vi "UHR-Fleezers Control (host) - 10.6.vi"() -> ()   [LabVIEW 2010] (continued)
        n1249 = control-ref of="Trap Delta (MHz)"() -> (w4746:refnum<vi>)
        n1250 = Equal?(x=w4746, y=w4747) -> (x = y?=w4745:bool)
        n1251 = case shown="False" "Oscillate Set 1" {
          tunnel: w4750 -> [w4770 _]
          tunnel: [w4769 w4773] -> w4749
          tunnel: w4748 -> [w4768 w4773]
          tunnel: w4745 -> [w4753 _]
          frame False {
            n1252 = local read "BD 1 Frequency 2 (MHz)"() -> (w4757:dbl)
            n1253 = local read "BD 1 Frequency 1 (MHz)"() -> (w4755:dbl)
            n1254 = Subtract(x=w4757, y="Trap Delta (MHz)") -> (x-y=w4754:dbl)
            n1255 = Select(t=w4754, s=w4753, f=w4755) -> (s? t:f=w4752:dbl)
            n1256 = local read "Y RF Frequency Limits (MHz)"() -> (w4758:T16)
            n1257 = local read "X RF Frequency Limits (MHz)"() -> (w4759:T16)
            n1258 = local read "BD 1 Frequency 3 (MHz)"() -> (w4771:dbl)
            n1259 = local write "BD 1 Frequency 1 (MHz)"(w4752) -> ()
            n1260 = local read "BD 2 Frequency 1 (MHz)"() -> (w4762:dbl)
            n1261 = local read "BD 2 Frequency 2 (MHz)"() -> (w4761:dbl)
            n1262 = local read "BD 2 Frequency 3 (MHz)"() -> (w4772:dbl)
            n1263 = call "set RF board frequency - interlace.vi"("Board 2 Frequency Limits"=w4758, "Board 1 Frequency Limits"=w4759, "error in"=w4768, "FPGA VI Reference In"=w4770, "Board 2 Frequency 3 (MHz)"=w4772, "Board 1 Frequency 3 (MHz)"=w4771, "Board 2 Frequency 2 (MHz)"=w4761, "Board 2 Frequency 1 (MHz)"=w4762, "Board 1 Frequency 2 (MHz)"=w4757, "Board 1 Frequency 1  (MHz)"=w4752) -> ("error out"=w4769:errorcluster)  [unwired: 1 out]
            n1264 = Subtract(x=w4762, y=w4761) -> (x-y=w4766:dbl)
            n1265 = Subtract(x=w4752, y=w4757) -> (x-y=w4767:dbl)
            n1266 = Square(x=w4766) -> (x^2=w4764:dbl)
            n1267 = Square(x=w4767) -> (x^2=w4765:dbl)
            n1268 = Add(x=w4765, y=w4764) -> (x+y=w4763:dbl)
            n1269 = Square Root(x=w4763) -> (sqrt(x)=w4760:dbl)
            n1270 = local write "Trap Delta (MHz)"(w4760) -> ()
            n1271 = property on="Initial delta (MHz)" class="DigNum (strict)"("Val(Sgnl)"=w4760) -> ()  [unwired: 2 in, 2 out]
          }
          frame True {
          }
        }
      }
      event "Round T1 X": Value Change {
        n1272 = event-data() -> ()  [unwired: 7 out]
        n1273 = local read "BD 1 Frequency 1 (MHz)"() -> (w4776:dbl)
        n1274 = Round To Nearest(number=w4776) -> (nearest integer value=w4775:dbl)
        n1275 = property on="BD 1 Frequency 1 (MHz)" class="DigNum (strict)"("Val(Sgnl)"=w4775) -> ()  [unwired: 2 in, 2 out]
      }
      event "Restart RF": Value Change {
        n1276 = event-data() -> ()  [unwired: 7 out]
        n1277 = xnode "Read/Write Control"("FPGA VI Reference In"=w4814, "error in"=w4809, "FPGA Controls  RF Box"=FALSE) -> ("FPGA VI Reference Out"=w4813:T20, "error out"=w4808:errorcluster)
        n1278 = local read "Y RF Amplitude Limits (%)"() -> (w4789:T16)
        n1279 = local read "X RF Amplitude Limits (%)"() -> (w4790:T16)
        n1280 = local read "X RF Frequency Limits (MHz)"() -> (w4792:T16)
        n1281 = local read "Y RF Frequency Limits (MHz)"() -> (w4791:T16)
        n1282 = xnode "Read/Write Control"("FPGA VI Reference In"=w4813, "error in"=w4808, "Direct RF Box  Communication"=TRUE) -> ("FPGA VI Reference Out"=w4812:T20, "error out"=w4807:errorcluster)
        n1283 = local read "BD 2 Frequency 3 (MHz)"() -> (w4799:dbl)
        n1284 = local read "BD 2 Frequency 2 (MHz)"() -> (w4800:dbl)
        n1285 = local read "BD 1 Frequency 3 (MHz)"() -> (w4803:dbl)
        n1286 = local read "BD 1 Frequency 1 (MHz)"() -> (w4804:dbl)
        n1287 = local read "BD 2 Frequency 1 (MHz)"() -> (w4801:dbl)
        n1288 = local read "BD 1 Frequency 2 (MHz)"() -> (w4802:dbl)
        n1289 = call "Initialize RF boards - interlace 3.vi"("error in"=w4807, "FPGA VI Reference In"=w4812) -> ("error out"=w4806:errorcluster, "FPGA VI Reference Out"=w4811:T20)
        n1290 = local read "BD 2 Amplitude 2 (%)"() -> (w4794:dbl)
        n1291 = local read "BD 2 Amplitude 1 (%)"() -> (w4795:dbl)
        n1292 = local read "BD 2 Amplitude 3 (%)"() -> (w4793:dbl)
        n1293 = local read "BD 1 Amplitude 3 (%)"() -> (w4798:dbl)
        n1294 = local read "BD 1 Amplitude 1 (%)"() -> (w4797:dbl)
        n1295 = local read "BD 1 Amplitude 2 (%)"() -> (w4796:dbl)
        n1296 = call "set RF board frequency - interlace.vi"("Board 2 Frequency Limits"=w4791, "Board 1 Frequency Limits"=w4792, "error in"=w4806, "FPGA VI Reference In"=w4811, "Board 2 Frequency 3 (MHz)"=w4799, "Board 1 Frequency 3 (MHz)"=w4803, "Board 2 Frequency 2 (MHz)"=w4800, "Board 2 Frequency 1 (MHz)"=w4801, "Board 1 Frequency 2 (MHz)"=w4802, "Board 1 Frequency 1  (MHz)"=w4804) -> ("error out"=w4805:errorcluster, "FPGA VI Reference Out"=w4810:T20)
        n1297 = call "set RF board amplitude - interlace.vi"("Board 2 Amplitude Limits"=w4789, "Board 1 Amplitude Limits"=w4790, "error in"=w4805, "FPGA VI Reference In"=w4810, "Board 2 Amplitude 3 (%)"=w4793, "Board 1 Amplitude 3 (%)"=w4798, "Board 2 Amplitude 2 (%)"=w4794, "Board 2 Amplitude 1 (%)"=w4795, "Board 1 Amplitude 2 (%)"=w4796, "Board 1 Amplitude 1 (%)"=w4797) -> ("error out"=w4782:errorcluster, "FPGA VI Reference Out"=w4786:T20)
        n1298 = xnode "Read/Write Control"("FPGA VI Reference In"=w4786, "error in"=w4782, "Direct RF Box  Communication"=FALSE) -> ("FPGA VI Reference Out"=w4785:T20, "error out"=w4784:errorcluster)
        n1299 = flat-sequence {
          tunnel: w4784 -> [w4815]
          tunnel: [w4815] -> w4783
          frame #0 {
            n1300 = Wait (ms)(milliseconds to wait=u32 50) -> ()  [unwired: 1 out]
          }
        }
        n1301 = xnode "Read/Write Control"("FPGA VI Reference In"=w4785, "error in"=w4783, "FPGA Controls  RF Box"=TRUE) -> ("error out"=w4778:errorcluster)  [unwired: 1 out]
        n1302 = property on="Restart RF" class="Bool (strict)"(error in=w4778, "Value"=FALSE ("Restart RF")) -> (error out=w4777:errorcluster)  [unwired: 1 in, 1 out]
      }
      event "Round T2 X": Value Change {
        n1303 = event-data() -> ()  [unwired: 7 out]
        n1304 = local read "BD 1 Frequency 2 (MHz)"() -> (w4970:dbl)
        n1305 = Round To Nearest(number=w4970) -> (nearest integer value=w4969:dbl)
        n1306 = property on="BD 1 Frequency 2 (MHz)" class="DigNum (strict)"("Val(Sgnl)"=w4969) -> ()  [unwired: 2 in, 2 out]
      }
      event "Stop All": Value Change {
        n1307 = event-data() -> ()  [unwired: 7 out]
        n1308 = local read "Stop All"() -> (w4972:bool)
      }
      event "Delayed Interlace Start": Value Change {
        n1309 = event-data() -> ()  [unwired: 7 out]
        n1310 = flat-sequence {
          frame #0 {
            n1311 = Multiply(x="Delay to Interlace (s)", y=1000.0) -> (x*y=w4975:dbl)
            n1312 = Wait (ms)(milliseconds to wait=w4975) -> ()  [unwired: 1 out]
          }
          frame #1 {
            n1313 = property on="Green laser mode" class="RadioBtnsControl (strict)"("Val(Sgnl)"=enum32{"Laser ON", "Laser OFF", "Interlace"}."Interlace" ("Value (Signaling)")) -> ()  [unwired: 2 in, 2 out]
          }
        }
      }
      event "BD 1 Amplitude 1 (%)", "BD 1 Amplitude 2 (%)", "BD 1 Amplitude 3 (%)", "BD 2 Amplitude 1 (%)", "BD 2 Amplitude 2 (%)", "BD 2 Amplitude 3 (%)", "Trap 1 ON", "Trap 2 ON", "Trap 3 ON", "Feedback On/Off", "All FB On/Off": Value Change {
        w4999 = i16 1 ("f")
        n1314 = event-data() -> ()  [unwired: 7 out]
        n1315 = local write "Trap 1 (ON/OFF)"("Trap 1 ON") -> ()
        n1316 = local write "Trap 2 (ON/OFF)"("Trap 2 ON") -> ()
        n1317 = Boolean To (0,1)(Boolean="Trap 3 ON") -> (0, 1=w5000:i16)
        n1318 = Boolean To (0,1)(Boolean="Trap 1 ON") -> (0, 1=w5001:i16)
        n1319 = Boolean To (0,1)(Boolean="Trap 2 ON") -> (0, 1=w5002:i16)
        n1320 = Select(t=w5002, s="Trap ON/OFF X or Y Amp?", f=w4999) -> (s? t:f=w4997:i16)
        n1321 = Select(t=w5001, s="Trap ON/OFF X or Y Amp?", f=w4999) -> (s? t:f=w4998:i16)
        n1322 = Select(t=w5000, s="Trap ON/OFF X or Y Amp?", f=w4999) -> (s? t:f=w4996:i16)
        n1323 = Select(t=w4999, s="Trap ON/OFF X or Y Amp?", f=w5002) -> (s? t:f=w4994:i16)
        n1324 = Select(t=w4999, s="Trap ON/OFF X or Y Amp?", f=w5001) -> (s? t:f=w4995:i16)
        n1325 = Select(t=w4999, s="Trap ON/OFF X or Y Amp?", f=w5000) -> (s? t:f=w4993:i16)
        n1326 = And(x="All FB On/Off", y="Feedback On/Off") -> (x .and. y?=w4991:cluster{"Set 1":bool, "Set 2":bool})
        n1327 = local read "BD 1 Amplitude 1 (%)"() -> (w5011:dbl)
        n1328 = local read "BD 1 Amplitude 2 (%)"() -> (w5010:dbl)
        n1329 = local read "BD 1 Amplitude 3 (%)"() -> (w5009:dbl)
        n1330 = Unbundle By Name(w4991) -> ("Set 1"=w4986:bool, "Set 2"=w4983:bool)
        n1331 = local read "Y RF Amplitude Limits (%)"() -> (w4979:T16)
        n1332 = local read "X RF Amplitude Limits (%)"() -> (w4980:T16)
        n1333 = local read "BD 2 Amplitude 1 (%)"() -> (w5012:dbl)
        n1334 = local read "BD 2 Amplitude 2 (%)"() -> (w5013:dbl)
        n1335 = local read "BD 2 Amplitude 3 (%)"() -> (w5014:dbl)
        n1336 = And(x="Trap 2 ON", y=w4983) -> (x .and. y?=w4981:bool)
        n1337 = And(x="Trap 1 ON", y=w4986) -> (x .and. y?=w4984:bool)
        n1338 = Multiply(x=w4998, y=w5011) -> (x*y=w5006:dbl)
        n1339 = Multiply(x=w5010, y=w4997) -> (x*y=w5004:dbl)
        n1340 = Multiply(x=w5009, y=w4996) -> (x*y=w5005:dbl)
        n1341 = Multiply(x=w5012, y=w4995) -> (x*y=w5015:dbl)
        n1342 = Multiply(x=w5013, y=w4994) -> (x*y=w5016:dbl)
        n1343 = Multiply(x=w5014, y=w4993) -> (x*y=w5017:dbl)
        n1344 = call "set RF board amplitude - interlace.vi"("Board 2 Amplitude Limits"=w4979, "Board 1 Amplitude Limits"=w4980, "error in"=w5007, "FPGA VI Reference In"=w5008, "Board 2 Amplitude 3 (%)"=w5017, "Board 1 Amplitude 3 (%)"=w5005, "Board 2 Amplitude 2 (%)"=w5016, "Board 2 Amplitude 1 (%)"=w5015, "Board 1 Amplitude 2 (%)"=w5004, "Board 1 Amplitude 1 (%)"=w5006) -> ("error out"=w4988:errorcluster, "FPGA VI Reference Out"=w4989:T20)
        n1345 = xnode "Read/Write Control"("FPGA VI Reference In"=w4989, "error in"=w4988, "FB On/Off Set 1"=w4984, "FB On/Off Set 2"=w4981) -> ("error out"=w4987:errorcluster)  [unwired: 1 out]
      }
      event "Load parameters": Value Change {
        n1346 = event-data() -> ()  [unwired: 7 out]
        n1347 = property on="Saved AOD Raster Scan Parameter Sets" class="Arr (strict)"() -> ("Index Values"=w5087:u32[])  [unwired: 2 in, 2 out]
        n1348 = Index Array(array=w5087, index=0) -> (element=w5084:u32)
        n1349 = local write "Load parameters"(FALSE ("Load parameters")) -> ()
        n1350 = Index Array(array="Saved AOD Raster Scan Parameter Sets", index=w5084) -> (element=w5083:T48)
        n1351 = Unbundle By Name(w5083) -> ("Scan Range AOD (nm) 2"=w5082:dbl, "Step Size AOD (nm) 2"=w5081:dbl, "Scan Speed AOD (nm/s) 2"=w5080:dbl, "Number of scans (AOD) 2"=w5079:u16)
        n1352 = flat-sequence {
          tunnel: w5082 -> [w5090]
          tunnel: w5081 -> [w5089]
          tunnel: w5080 -> [w5088]
          tunnel: w5079 -> [w5091]
          frame #0 {
            n1353 = local write "Scan Speed (nm/s)"(w5088) -> ()
            n1354 = local write "Scan Range (nm)"(w5090) -> ()
            n1355 = local write "Step Size (nm)"(w5089) -> ()
          }
          frame #1 {
            n1356 = property on="Number of F/B Scans (AOD)" class="DigNum (strict)"("Val(Sgnl)"=w5091) -> ()  [unwired: 2 in, 2 out]
          }
        }
      }
      event "Trap 1 (ON/OFF)", "Trap 2 (ON/OFF)": Value Change {
        n1357 = event-data() -> ()  [unwired: 7 out]
        n1358 = property on="Trap 2 ON" class="Bool (strict)"("Val(Sgnl)"="Trap 2 (ON/OFF)") -> ()  [unwired: 2 in, 2 out]
        n1359 = property on="Trap 1 ON" class="Bool (strict)"("Val(Sgnl)"="Trap 1 (ON/OFF)") -> ()  [unwired: 2 in, 2 out]
      }
      event "DIO count 1 (ticks)", "DIO count 2 (ticks)", "DIO count 3 (ticks)", "Interlace", "Number Interlace Sets", "Not-Interlacing Set": Value Change {
        n1360 = event-data() -> ()  [unwired: 7 out]
        n1361 = local read "DIO count 3 (ticks)"() -> (w5104:u32)
        n1362 = local read "DIO count 1 (ticks)"() -> (w5106:u32)
        n1363 = local read "DIO count 2 (ticks)"() -> (w5105:u32)
        n1364 = To Unsigned Byte Integer(number="Not-Interlacing Set") -> (unsigned 8bit integer=w5095:u8)
        n1365 = Add(x=w5095, y=u8 1) -> (x+y=w5099:u8)
        n1366 = xnode "Read/Write Control"("FPGA VI Reference In"=w5110, "error in"=w5108, "DIO count 1 (ticks)"=w5106, "DIO count 2 (ticks)"=w5105, "DIO count 3 (ticks)"=w5104, "Interlace ON/OFF"="Interlace", "Number Interlace Cycles"="Number Interlace Sets", "Interlace Off Parameters"=w5099) -> ("error out"=w5109:errorcluster)  [unwired: 1 out]
        n1367 = Build Array(w5106, w5105, w5104) -> (w5097:u32[])
        n1368 = Split 1D Array(array=w5097, index="Number Interlace Sets") -> (first subarray=w5107:u32[])  [unwired: 1 out]
        n1369 = Index Array(array=w5097, index=w5095) -> (element=w5096:u32)
        n1370 = Add Array Elements(numeric array=w5107) -> (sum=w5101:u32)
        n1371 = Select(t=w5101, s="Interlace", f=w5096) -> (s? t:f=→"Total Counts (ticks)":u32)
      }
      event "Reset Feedback": Value Change {
        n1372 = event-data() -> ()  [unwired: 7 out]
        n1373 = Unbundle By Name("Reset Feedback") -> ("Set 1"=w5252:bool, "Set 2"=w5251:bool)
        n1374 = xnode "Read/Write Control"("FPGA VI Reference In"=w5254, "error in"=w5249, "FB Reset Set 1"=w5252, "FB Reset Set 2"=w5251) -> ("error out"=w5250:errorcluster)  [unwired: 1 out]
      }
      event "PID Gains": Value Change {
        n1375 = event-data() -> ()  [unwired: 7 out]
        n1376 = Unbundle By Name("PID Gains") -> ("Set 1"=w5317:T14, "Set 2"=w5316:T14)
        n1377 = xnode "Read/Write Control"("FPGA VI Reference In"=w5318, "error in"=w5314, "FB Gains Set 1"=w5317, "FB Gains Set 2"=w5316) -> ("error out"=w5315:errorcluster)  [unwired: 1 out]
      }
      event "AI2 to Setpoint", "Trap Intensity\nSetpoints (V)": Value Change {
        n1378 = event-data() -> ()  [unwired: 7 out]
        n1379 = xnode "Read/Write Control"("FPGA VI Reference In"=w5393, "error in"=w5389) -> ("FPGA VI Reference Out"=w5392:T20, "error out"=w5391:errorcluster, "AI2 Y Sum Set 1"=w5400:i16, "AI2 Y Sum Set 2"=w5399:i16)
        n1380 = Cluster To Array(cluster="AI2 to Setpoint") -> (array=w5403:bool[])
        n1381 = local read "AI2 (V)"() -> (w5401:cluster{"Set 1":dbl, "Set 2":dbl})
        n1382 = Or Array Elements(Boolean array=w5403) -> (logical OR=w5404:bool)
        n1383 = Bundle By Name(cluster=w5401, "Set 1"=w5400, "Set 2"=w5399) -> (w5398:cluster{"Set 1":dbl, "Set 2":dbl})
        n1384 = Divide(x=w5398, y=3276.7) -> (x/y=w5397:cluster{"Set 1":dbl, "Set 2":dbl})
        "AI2 (V)" <- w5397
        n1385 = case shown="True" w5404 {
          tunnel: [w5468 w5485] -> w5396
          tunnel: "AI2 to Setpoint" -> [_ w5481]
          tunnel: "Trap Intensity\nSetpoints (V)" -> [w5469 w5484]
          tunnel: w5397 -> [_ w5478]
          frame False {
            n1386 = Multiply(x=3276.7, y=w5469) -> (x*y=w5470:cluster{"Set 1":dbl, "Set 2":dbl})
            n1387 = To Word Integer(number=w5470) -> (16bit integer=w5468:cluster{"Set 1":i16, "Set 2":i16})
          }
          frame True {
            n1388 = Unbundle By Name(w5478) -> ("Set 1"=w5477:dbl, "Set 2"=w5476:dbl)
            n1389 = Unbundle By Name(w5484) -> ("Set 1"=w5483:dbl, "Set 2"=w5482:dbl)
            n1390 = Unbundle By Name(w5481) -> ("Set 1"=w5480:bool, "Set 2"=w5479:bool)
            n1391 = Select(t=w5477, s=w5480, f=w5483) -> (s? t:f=w5475:dbl)
            n1392 = Select(t=w5476, s=w5479, f=w5482) -> (s? t:f=w5474:dbl)
            n1393 = Bundle By Name(cluster=w5484, "Set 1"=w5475, "Set 2"=w5474) -> (w5472:cluster{"Set 1":dbl, "Set 2":dbl})
            n1394 = local write "Trap Intensity\nSetpoints (V)"(w5472) -> ()
            n1395 = Multiply(x=3276.7, y=w5472) -> (x*y=w5473:cluster{"Set 1":dbl, "Set 2":dbl})
            n1396 = To Word Integer(number=w5473) -> (16bit integer=w5485:cluster{"Set 1":i16, "Set 2":i16})
          }
        }
        n1397 = Unbundle By Name(w5396) -> ("Set 1"=w5395:i16, "Set 2"=w5394:i16)
        n1398 = xnode "Read/Write Control"("FPGA VI Reference In"=w5392, "error in"=w5391, "FB Setpoint Set 1"=w5395, "FB Setpoint Set 2"=w5394) -> ("error out"=w5390:errorcluster)  [unwired: 1 out]
      }
      event "Invert GI": Value Change {
        n1399 = event-data() -> ()  [unwired: 7 out]
        n1400 = xnode "Read/Write Control"("FPGA VI Reference In"=w5547, "error in"=w5545, "Invert GI"="Invert GI", "Invert GI 2"="Invert GI") -> ("error out"=w5546:errorcluster)  [unwired: 1 out]
      }
      event "Green FB Setpoint (mV)", "Green FB Gains", "Green FB On/Off", "Current When FB OFF (%)", "Green int current ON count adj": Value Change {
        n1401 = event-data() -> ()  [unwired: 7 out]
        n1402 = local read "Green FB Setpoint (mV)"() -> (w5613:dbl)
        n1403 = local read "Current When FB OFF (%)"() -> (w5616:dbl)
        n1404 = Multiply(x=w5613, y=3.2767) -> (x*y=w5612:dbl)
        n1405 = Multiply(x=w5616, y=655.35) -> (x*y=w5617:dbl)
        n1406 = To Unsigned Word Integer(number=w5617) -> (unsigned 16bit integer=w5615:u16)
        n1407 = local read "Green int current ON count adj"() -> (w5620:u32)
        n1408 = local read "Green FB Gains"() -> (w5619:T14)
        n1409 = local read "Green Laser ON/Interlacing"() -> (w5610:bool)
        n1410 = local read "Green laser mode"() -> (w5609:enum32{"Laser ON", "Laser OFF", "Interlace"})
        n1411 = local read "Green FB On/Off"() -> (w5621:bool)
        n1412 = Equal?(x=w5609, y=enum32{"Laser ON", "Laser OFF", "Interlace"}."Interlace") -> (x = y?=w5607:bool)
        n1413 = Compound Arithmetic op=AND(w5607, w5621, w5610) -> (w5611:bool)
        n1414 = xnode "Read/Write Control"("FPGA VI Reference In"=w5624, "error in"=w5623, "Green FB Setpoint"=w5612, "Green FB On/Off"=w5611, "Current Out"=w5615, "Green int current ON count adj"=w5620, "Green FB Gains"=w5619) -> ("error out"=w5622:errorcluster)  [unwired: 1 out]
      }
      event "Green laser mode", "Green Laser ON/Interlacing": Value Change {
        n1415 = event-data() -> ()  [unwired: 7 out]
        n1416 = case shown="True" "Green Laser ON/Interlacing" {
          tunnel: "Green laser mode" -> [_ w5762]
          tunnel: [enum32{"Laser ON", "Laser OFF", "Interlace"}."Laser OFF" ("Green laser mode") w5762] -> w5750
          tunnel: [FALSE w5758] -> w5749
          frame False {
          }
          frame True {
            n1417 = local read "Green FB On/Off"() -> (w5759:bool)
            n1418 = Equal?(x=w5762, y=enum32{"Laser ON", "Laser OFF", "Interlace"}."Interlace") -> (x = y?=w5760:bool)
            n1419 = And(x=w5760, y=w5759) -> (x .and. y?=w5758:bool)
          }
        }
        n1420 = xnode "Read/Write Control"("FPGA VI Reference In"=w5755, "error in"=w5753, "Operating Mode"=w5750, "Operating Mode 2"=w5750, "Green FB On/Off"=w5749) -> ("error out"=w5754:errorcluster)  [unwired: 1 out]
      }
      event "Use mouse to move stage\n(press mouse wheel to quit)": Value Change {
        n1421 = event-data() -> ()  [unwired: 7 out]
      }
      event "- phase (APD 1 Gate)", "+ phase (APD 1 Gate)": Value Change {
        n1422 = event-data() -> ()  [unwired: 7 out]
        n1423 = local read "Phase Adj. (APD 1 Gate)"() -> (w5841:i16)
        n1424 = Negate(x=w5841) -> (-x=w5849:i16)
        n1425 = Select(t=w5849, s="- phase (APD 1 Gate)", f=w5841) -> (s? t:f=w5848:i16)
        n1426 = Or(x="- phase (APD 1 Gate)", y="+ phase (APD 1 Gate)") -> (x .or. y?=w5844:bool)
        n1427 = xnode "Read/Write Control"("FPGA VI Reference In"=w5851, "error in"=w5850, "Phase count adjustment (APD 1 Gate)"=w5848) -> ("FPGA VI Reference Out"=w5846:T20, "error out"=w5847:errorcluster)
        n1428 = xnode "Read/Write Control"("FPGA VI Reference In"=w5846, "error in"=w5847, "+ phase (APD 1 Gate)"=w5844) -> ("error out"=w5845:errorcluster)  [unwired: 1 out]
      }
      event "+ phase (APD 2 Gate)", "- phase (APD 2 Gate)": Value Change {
        n1429 = event-data() -> ()  [unwired: 7 out]
        n1430 = local read "Phase Adj. (APD 2 Gate)"() -> (w5927:i16)
        n1431 = Negate(x=w5927) -> (-x=w5935:i16)
        n1432 = Select(t=w5935, s="- phase (APD 2 Gate)", f=w5927) -> (s? t:f=w5934:i16)
        n1433 = Or(x="- phase (APD 2 Gate)", y="+ phase (APD 2 Gate)") -> (x .or. y?=w5930:bool)
        n1434 = xnode "Read/Write Control"("FPGA VI Reference In"=w5937, "error in"=w5936, "Phase count adjustment (APD 2 Gate)"=w5934) -> ("FPGA VI Reference Out"=w5932:T20, "error out"=w5933:errorcluster)
        n1435 = xnode "Read/Write Control"("FPGA VI Reference In"=w5932, "error in"=w5933, "+ phase (APD 2 Gate)"=w5930) -> ("error out"=w5931:errorcluster)  [unwired: 1 out]
      }
      event "Phase Adj. (APD Acq)", "+ phase (APD Acq)", "- phase (APD Acq)": Value Change {
        n1436 = event-data() -> ()  [unwired: 7 out]
        n1437 = local read "Phase Adj. (APD Acq)"() -> (w6015:i16)
        n1438 = Negate(x=w6015) -> (-x=w6021:i16)
        n1439 = Select(t=w6021, s="+ phase (APD Acq)", f=w6015) -> (s? t:f=w6020:i16)
        n1440 = Or(x="+ phase (APD Acq)", y="- phase (APD Acq)") -> (x .or. y?=w6016:bool)
        n1441 = xnode "Read/Write Control"("FPGA VI Reference In"=w6023, "error in"=w6022, "Phase Count Adjustment (APD Acq)"=w6020) -> ("FPGA VI Reference Out"=w6018:T20, "error out"=w6019:errorcluster)
        n1442 = xnode "Read/Write Control"("FPGA VI Reference In"=w6018, "error in"=w6019, "+ phase (APD Acq)"=w6016) -> ("error out"=w6017:errorcluster)  [unwired: 1 out]
      }
      event "Phase adj. (GI)", "+ phase (GI)", "- phase (GI)": Value Change {
        n1443 = event-data() -> ()  [unwired: 7 out]
        n1444 = Negate(x="Phase adj. (GI)") -> (-x=w6107:i16)
        n1445 = Select(t=w6107, s="+ phase (GI)", f="Phase adj. (GI)") -> (s? t:f=w6106:i16)
        n1446 = Or(x="+ phase (GI)", y="- phase (GI)") -> (x .or. y?=w6102:bool)
        n1447 = xnode "Read/Write Control"("FPGA VI Reference In"=w6109, "error in"=w6108, "Phase count adjustment (GI)"=w6106) -> ("FPGA VI Reference Out"=w6104:T20, "error out"=w6105:errorcluster)
        n1448 = xnode "Read/Write Control"("FPGA VI Reference In"=w6104, "error in"=w6105, "+ phase (GI)"=w6102) -> ("error out"=w6103:errorcluster)  [unwired: 1 out]
      }
      event "Phase adj. (GI) 2", "+ phase (GI) 2", "- phase (GI) 2": Value Change {
        n1449 = event-data() -> ()  [unwired: 7 out]
        n1450 = Negate(x="Phase adj. (GI) 2") -> (-x=w6193:i16)
        n1451 = Select(t=w6193, s="+ phase (GI) 2", f="Phase adj. (GI) 2") -> (s? t:f=w6192:i16)
        n1452 = Or(x="+ phase (GI) 2", y="- phase (GI) 2") -> (x .or. y?=w6188:bool)
        n1453 = xnode "Read/Write Control"("FPGA VI Reference In"=w6195, "error in"=w6194, "Phase count adjustment (GI) 2"=w6192) -> ("FPGA VI Reference Out"=w6190:T20, "error out"=w6191:errorcluster)
        n1454 = xnode "Read/Write Control"("FPGA VI Reference In"=w6190, "error in"=w6191, "+ phase (GI) 2"=w6188) -> ("error out"=w6189:errorcluster)  [unwired: 1 out]
      }
      event "Phase adj. (Green FB)", "- phase (Green FB)", "+ phase (Green FB)": Value Change {
        n1455 = event-data() -> ()  [unwired: 7 out]
        n1456 = Negate(x="Phase adj. (Green FB)") -> (-x=w6279:i16)
        n1457 = Select(t=w6279, s="+ phase (Green FB)", f="Phase adj. (Green FB)") -> (s? t:f=w6278:i16)
        n1458 = Or(x="+ phase (Green FB)", y="- phase (Green FB)") -> (x .or. y?=w6274:bool)
        n1459 = xnode "Read/Write Control"("FPGA VI Reference In"=w6281, "error in"=w6280, "Phase count adjustment (Green FB)"=w6278) -> ("FPGA VI Reference Out"=w6276:T20, "error out"=w6277:errorcluster)
        n1460 = xnode "Read/Write Control"("FPGA VI Reference In"=w6276, "error in"=w6277, "+ phase (Green FB)"=w6274) -> ("error out"=w6275:errorcluster)  [unwired: 1 out]
      }
      event "Invert APD Gate", "APD Gate ON Count", "APD Gate OFF Count", "APD Gate", "APD Integration Time (s)", "APD 1 AO Mult.", "APD 2 AO Mult.": Value Change {
        n1461 = event-data() -> ()  [unwired: 7 out]
        n1462 = local read "APD Integration Time (s)"() -> (w6357:dbl)
        n1463 = local read "APD Gate ON Count"() -> (w6370:u32)
        n1464 = local read "APD Gate OFF Count"() -> (w6369:u32)
        n1465 = local read "Invert APD Gate"() -> (w6371:bool)
        n1466 = local read "APD Gate"() -> (w6368:enum32{"ON", "OFF", "Interlace"})
        n1467 = Multiply(x=w6357, y=40000000.0) -> (x*y=w6366:dbl)
        n1468 = Reciprocal(x=w6357) -> (1/x=→"APD Acq Rate (Hz)":dbl)
        n1469 = To Unsigned Long Integer(number=w6366) -> (unsigned 32bit integer=w6365:u32)
        n1470 = local read "DMA Update Period (s)"() -> (w6358:dbl)
        n1471 = Divide(x=w6358, y=w6357) -> (x/y=w6361:dbl)
        n1472 = local read "APD 1 AO Mult."() -> (w6363:i16)
        n1473 = local read "APD 2 AO Mult."() -> (w6362:i16)
        n1474 = Multiply(x=2.0, y=w6361) -> (x*y=w6360:dbl)
        n1475 = local write "APD Samples/FIFO Acq."(w6361) -> ()
        n1476 = local write "APD Elements/DMA read"(w6360) -> ()
        n1477 = xnode "Read/Write Control"("FPGA VI Reference In"=w6374, "error in"=w6373, "Invert APD Gate"=w6371, "APD Gate ON Count"=w6370, "APD Gate OFF Count"=w6369, "APD Acq Rate Count"=w6365, "APD Gate Operating Mode"=w6368, "APD 1 AO scale factor"=w6363, "APD 2 AO scale factor"=w6362) -> ("error out"=w6372:errorcluster)  [unwired: 1 out]
      }
      event "GI Frequency, ON count", "Green FB Count", "GI Frequency, OFF count": Value Change {
        n1478 = event-data() -> ()  [unwired: 7 out]
        n1479 = xnode "Read/Write Control"("FPGA VI Reference In"=w6538, "error in"=w6536, "Green interlace ON count"="GI Frequency, ON count", "Green interlace OFF count"="GI Frequency, OFF count", "Green interlace ON count 2"="GI Frequency, ON count", "Green interlace OFF count 2"="GI Frequency, OFF count", "Green FB Count"="Green FB Count") -> ("error out"=w6537:errorcluster)  [unwired: 1 out]
      }
      event "Number of F/B Scans (AOD)", "Scan Speed (nm/s)", "Scan BD", "Initial delta (MHz)", "Step Size (nm)", "Scan Range (nm)": Value Change {
        n1480 = event-data() -> ()  [unwired: 7 out]
        n1481 = local read "BD 1 Frequency 1 (MHz)"() -> (w6701:dbl)
        n1482 = local read "AOM X Cal (nm/MHz)"() -> (w6693:dbl)
        n1483 = local read "X RF Frequency Limits (MHz)"() -> (w6705:T16)
        n1484 = local read "Y RF Frequency Limits (MHz)"() -> (w6702:T16)
        n1485 = local read "BD 2 Frequency 1 (MHz)"() -> (w6707:dbl)
        n1486 = Negate(x="Scan Range (nm)") -> (-x=w6671:dbl)
        n1487 = Divide(x=w6671, y=w6693) -> (x/y=w6675:dbl)
        n1488 = Select(t=w6705, s="Scan BD", f=w6702) -> (s? t:f=w6704:T16)
        n1489 = Select(t=w6701, s="Scan BD", f=w6707) -> (s? t:f=w6706:dbl)
        n1490 = Unbundle By Name(w6704) -> ("Maximum"=w6713:dbl, "Minimum"=w6712:dbl)
        n1491 = Add(x=w6675, y=w6706) -> (x+y=w6710:dbl)
        n1492 = Divide(x=w6671, y="Step Size (nm)") -> (x/y=w6690:dbl)
        n1493 = Divide(x="Step Size (nm)", y=w6693) -> (x/y=w6699:dbl)
        n1494 = Absolute Value(x=w6690) -> (abs(x)=w6674:dbl)
        n1495 = Sign(1:w6671) -> (0:w6672:dbl)
        n1496 = In Range and Coerce(upper limit=w6713, x=w6710, lower limit=w6712) -> (coerced(x)=w6709:dbl, In Range?=w6711:bool)
        n1497 = To Unsigned Quad Integer(1:w6674) -> (0:w6689:u64)
        "Scan steps (AOD)" <- w6689
        n1498 = call "IR AOM freq to word.vi"("Frequency In (MHz)"=w6699) -> ("Frequency Word Out (double)"=w6696:dbl)
        n1499 = Multiply(x=w6672, y=w6696) -> (x*y=w6673:dbl)
        n1500 = Subtract(x=w6710, y=w6709) -> (x-y=w6708:dbl)
        n1501 = To Quad Integer(1:w6673) -> (0:w6695:i64)
        "Incr. int (AOD)" <- w6695
        n1502 = Subtract(x=w6675, y=w6708) -> (x-y=w6694:dbl)
        "Scan Range (MHz)" <- w6694
        n1503 = Select(t=w6675, s=w6711, f=w6694) -> (s? t:f=w6714:dbl)
        n1504 = Multiply(x=w6694, y=w6693) -> (x*y=w6692:dbl)
        n1505 = Decrement(x=w6689) -> (x-1=w6741:u64)
        n1506 = Negate(x=w6692) -> (-x=w6688:dbl)
        n1507 = local write "Scan Range (nm)"(w6688) -> ()
        n1508 = Divide(x=w6714, y=w6741) -> (x/y=w6698:dbl)
        "Scan Increment (MHz)" <- w6698
        n1509 = call "IR AOM freq to word.vi"("Frequency In (MHz)"=w6698) -> ("Frequency Word Out (double)"=w6697:dbl)
        n1510 = Divide(x="Step Size (nm)", y="Scan Speed (nm/s)") -> (x/y=w6685:dbl)
        n1511 = To Quad Integer(1:w6697) -> ()  [unwired: 1 out]
        n1512 = local read "Number Interlace Sets"() -> (w6669:u8)
        n1513 = local read "AI Count (ticks)"() -> (w6670:u32)
        n1514 = local read "Total Counts (ticks)"() -> (w6668:u32)
        n1515 = local read "# Samples/trap"() -> (w6700:u32)
        n1516 = Multiply(x=w6670, y=w6669) -> (x*y=w6667:u32)
        n1517 = Divide(x=w6668, y=w6667) -> (x/y=w6666:dbl)
        n1518 = local read "AOM X Cal (nm/MHz)"() -> (w6656:dbl)
        n1519 = Select(t=w6701, s="Scan BD", f=w6707) -> (s? t:f=w6738:dbl)
        "Initial freq. (MHz)" <- w6738
        n1520 = Add(x=w6714, y=w6738) -> (x+y=→"Final freq. (MHz)":dbl)
        n1521 = Divide(x=w6668, y=40000000.0) -> (x/y=w6684:dbl)
        n1522 = Divide(x=w6685, y=w6684) -> (x/y=w6683:dbl)
        n1523 = To Unsigned Quad Integer(1:w6683) -> (0:w6658:u64)
        n1524 = Quotient & Remainder(x=w6658, y=u64 2) -> (x-y*floor(x/y)=w6662:u64)  [unwired: 1 out]
        n1525 = Equal?(x=w6662, y=u64 0) -> (x = y?=w6660:bool)
        n1526 = Decrement(x=w6658) -> (x-1=w6659:u64)
        n1527 = Select(t=w6658, s=w6660, f=w6659) -> (s? t:f=w6657:u64)
        "Cycles/step (AOD)" <- w6657
        n1528 = xnode "Read/Write Control"("FPGA VI Reference In"=w6749, "error in"=w6748, "Scan steps"=w6689, "Number of scans"="Number of F/B Scans (AOD)", "Cycles per step"=w6657, "Scan freq.  increment"=w6695, "Scan BD"="Scan BD") -> ("error out"=w6747:errorcluster)  [unwired: 1 out]
        n1529 = Multiply(x=w6689, y=w6657) -> (x*y=w6742:u64)
        n1530 = Multiply(x=w6742, y=u64 2) -> (x*y=w6665:u64)
        n1531 = Multiply(x=w6666, y=w6665) -> (x*y=w6664:dbl)
        "Data points/scan (f/b)" <- w6664
        n1532 = Multiply(x=w6664, y="Number of F/B Scans (AOD)") -> (x*y=w6745:dbl)
        "Data points/scans" <- w6745
        n1533 = Divide(x=w6745, y=w6700) -> (x/y=→"N sets should be saved":dbl)
        n1534 = Multiply(x=w6742, y=w6684) -> (x*y=w6682:dbl)
        "Time/Scan (s) (AOD)" <- w6682
        n1535 = Select(t=w6714, s="Scan BD", f=0.0) -> (s? t:f=w6739:dbl)
        n1536 = Select(t=0.0, s="Scan BD", f=w6714) -> (s? t:f=w6735:dbl)
        n1537 = local read "BD 2 Frequency 2 (MHz)"() -> (w6731:dbl)
        n1538 = local read "BD 1 Frequency 2 (MHz)"() -> (w6734:dbl)
        n1539 = Add(x=w6735, y=w6707) -> (x+y=w6732:dbl)
        n1540 = Add(x=w6701, y=w6739) -> (x+y=w6733:dbl)
        n1541 = Multiply(x=w6682, y=2.0) -> (x*y=w6681:dbl)
        n1542 = Multiply(x=w6681, y="Number of F/B Scans (AOD)") -> (x*y=w6678:dbl)
        n1543 = Divide(x=w6678, y=60.0) -> (x/y=→"Time to Finish All (min)":dbl)
        n1544 = Add(x="Trap 2 Bead Size (nm)", y="Trap 1 Bead Size (nm)") -> (x+y=w6721:dbl)
        n1545 = Divide(x=w6721, y=2.0) -> (x/y=w6716:dbl)
        n1546 = local read "Initial delta (MHz)"() -> (w6718:dbl)
        n1547 = Subtract(x=w6732, y=w6731) -> (x-y=w6729:dbl)
        n1548 = Subtract(x=w6733, y=w6734) -> (x-y=w6730:dbl)
        n1549 = Square(x=w6729) -> (x^2=w6728:dbl)
        n1550 = Square(x=w6730) -> (x^2=w6727:dbl)
        n1551 = Add(x=w6727, y=w6728) -> (x+y=w6726:dbl)
        n1552 = Square Root(x=w6726) -> (sqrt(x)=w6725:dbl)
        "Final delta (MHz)" <- w6725
        n1553 = Multiply(x=w6656, y=w6725) -> (x*y=w6724:dbl)
        n1554 = Multiply(x=w6718, y=w6656) -> (x*y=w6717:dbl)
        n1555 = Subtract(x=w6717, y=w6716) -> (x-y=→"Initial sep (nm)":dbl)
        n1556 = Subtract(x=w6724, y=w6716) -> (x-y=→"Final sep (nm)":dbl)
      }
      event "Freq or Amp switch first", "Swap F1 and F2", "Freq switch delay", "Amp switch delay": Value Change {
        n1557 = event-data() -> ()  [unwired: 7 out]
        n1558 = local read "Freq or Amp switch first"() -> (w6886:bool)
        n1559 = local read "Amp switch delay"() -> (w6887:u16)
        n1560 = local read "Freq switch delay"() -> (w6889:u16)
        n1561 = local read "Swap F1 and F2"() -> (w6888:bool)
        n1562 = xnode "Read/Write Control"("FPGA VI Reference In"=w6892, "error in"=w6891, "Freq switch delay"=w6889, "Swap F1 and F2"=w6888, "Amp switch delay"=w6887, "Freq or Amp switch first"=w6886) -> ("error out"=w6890:errorcluster)  [unwired: 1 out]
      }
      event "Scan steps (MCL)", "Number of scans (MCL)", "Scan Range (V)\n(of steps)", "2D or 1D Scan", "N APD Samp/step", "Fast Scan Dir", "Continuous MCL Scanning", "Scan lines (y)": Value Change {
        w6993 = 32767.0 ("y")
        n1563 = event-data() -> ()  [unwired: 7 out]
        n1564 = Select(t="Scan lines (y)", s="2D or 1D Scan", f="Number of scans (MCL)") -> (s? t:f=w6998:u64)
        n1565 = Decrement(x="Scan steps (MCL)") -> (x-1=w7014:u64)
        n1566 = Divide(x="Scan Range (V)\n(of steps)", y=w7014) -> (x/y=w7013:dbl)
        "Desired Scan Incr (V)" <- w7013
        n1567 = local read "APD Integration Time (s)"() -> (w7006:dbl)
        n1568 = Multiply(x=w7013, y=w6993) -> (x*y=w7022:dbl)
        n1569 = Divide(x=w7022, y=10.0) -> (x/y=w7012:dbl)
        "Desired incr (int)" <- w7012
        n1570 = local read "Update Count (MCL)"() -> (w7018:u32)
        n1571 = Round Toward -Infinity(1:w7012) -> (0:w7021:dbl)
        n1572 = To Word Integer(number=w7021) -> (16bit integer=w6996:i16)
        "Actual Incr. int (MCL)" <- w6996
        n1573 = Multiply(x=w7006, y=40000000.0) -> (x*y=w7019:dbl)
        n1574 = Divide(x=w7019, y=w7018) -> (x/y=w7017:dbl)
        n1575 = Multiply(x=i16 10, y=w6996) -> (x*y=w6994:i16)
        n1576 = Multiply(x="N APD Samp/step", y=w7017) -> (x*y=w7016:dbl)
        "Cycles/step (MCL)" <- w7016
        n1577 = Divide(x=w6994, y=w6993) -> (x/y=→"Actual MCL Inc (V)":dbl)
        n1578 = Multiply(x="N APD Samp/step", y="Scan steps (MCL)") -> (x*y=w7008:dbl)
        n1579 = local read "APD Samples/FIFO Acq."() -> (w7005:dbl)
        n1580 = Multiply(x=w7008, y=u64 2) -> (x*y=w7007:dbl)
        "Data points/scan (f+b)" <- w7007
        n1581 = Multiply(x=w7007, y=w6998) -> (x*y=w7025:dbl)
        "Data points/scans (MCL)" <- w7025
        n1582 = Multiply(x=w7006, y=w7007) -> (x*y=w6999:dbl)
        "Time/f+b scan (s) (MCL)" <- w6999
        n1583 = Divide(x=w7025, y=w7005) -> (x/y=→"N sets should be saved (MCL)":dbl)
        n1584 = Multiply(x=w6999, y=w6998) -> (x*y=→"Total Time (s)":dbl)
        n1585 = Not(x="Fast Scan Dir") -> (.not. x?=w7003:bool)
        n1586 = xnode "Read/Write Control"("FPGA VI Reference In"=w7029, "error in"=w7028, "Scan steps (MCL)"="Scan steps (MCL)", "Number of scans (MCL)"=w6998, "Cycles per step (MCL)"=w7016, "Scan freq.  increment (MCL)"=w6996, "1D or 2D Scan?"="2D or 1D Scan", "MCL Scan Axis"=w7003, "Cont. Scan (MCL)"="Continuous MCL Scanning") -> ("error out"=w7027:errorcluster)  [unwired: 1 out]
      }
      event Key Down {
        n1587 = event-data() -> ("VKey"=w7203:T49)  [unwired: 10 out]
        n1588 = local read "z nudge increment (um)"() -> (w7202:dbl)
        n1589 = case shown="\"F5\"" w7203 {
          tunnel: "lateral step size (mm)" -> [w7206 w7211 w7216 w7224 _ _ _ _ _ _ _ _ _ _ _ _ _ _ _ _ _ _ _ _ _ _ _ _ _ _ _ _ _ _ _ _ _ _ _ _ _ _ _ _ _ _ _ _ _ _ _ _ _ _ _ _]
          tunnel: w7202 -> [_ _ _ _ w7227 w7234 _ _ _ _ _ _ _ _ _ _ _ _ _ _ _ _ _ _ _ _ _ _ _ _ _ _ _ _ _ _ _ _ _ _ _ _ _ _ _ _ _ _ _ _ _ _ _ _ _ _]
          frame "Up" {
            w7208 = 0.0 ("element")
            n1590 = Negate(x=w7206) -> (-x=w7205:dbl)
            n1591 = Build Array(w7208, w7205, w7208) -> (w7207:dbl[])
            n1592 = call "CONEX_FUNCTIONAL_GLOBAL.vi"("Axis"=enum16{"X", "Y", "Z", "XY", "XZ", "YZ", "XYZ"}."Y", "Position"=w7207, "Command"=T23."REL MOVE") -> ()  [unwired: 6 in, 3 out]
          }
          frame "Down" {
            w7213 = 0.0 ("element")
            n1593 = Build Array(w7213, w7211, w7213) -> (w7212:dbl[])
            n1594 = call "CONEX_FUNCTIONAL_GLOBAL.vi"("Axis"=enum16{"X", "Y", "Z", "XY", "XZ", "YZ", "XYZ"}."Y", "Position"=w7212, "Command"=T23."REL MOVE") -> ()  [unwired: 6 in, 3 out]
          }
          frame "Left" {
            w7217 = 0.0 ("element")
            n1595 = Build Array(w7216, w7217, w7217) -> (w7218:dbl[])
            n1596 = call "CONEX_FUNCTIONAL_GLOBAL.vi"("Axis"=enum16{"X", "Y", "Z", "XY", "XZ", "YZ", "XYZ"}."X", "Position"=w7218, "Command"=T23."REL MOVE") -> ()  [unwired: 6 in, 3 out]
          }
          frame "Right" {
            w7222 = 0.0 ("element")
            n1597 = Negate(x=w7224) -> (-x=w7223:dbl)
            n1598 = Build Array(w7223, w7222, w7222) -> (w7221:dbl[])
            n1599 = call "CONEX_FUNCTIONAL_GLOBAL.vi"("Axis"=enum16{"X", "Y", "Z", "XY", "XZ", "YZ", "XYZ"}."X", "Position"=w7221, "Command"=T23."REL MOVE") -> ()  [unwired: 6 in, 3 out]
          }
          frame "PageUp" {
            w7231 = 0.0 ("element")
            n1600 = Divide(x=w7227, y=1000.0) -> (x/y=w7229:dbl)
            n1601 = Build Array(w7231, w7231, w7229) -> (w7230:dbl[])
            n1602 = call "CONEX_FUNCTIONAL_GLOBAL.vi"("Axis"=enum16{"X", "Y", "Z", "XY", "XZ", "YZ", "XYZ"}."Z", "Position"=w7230, "Command"=T23."REL MOVE") -> ()  [unwired: 6 in, 3 out]
          }
          frame "PageDown" {
            w7238 = 0.0 ("element")
            n1603 = Divide(x=w7234, y=-1000.0) -> (x/y=w7236:dbl)
            n1604 = Build Array(w7238, w7238, w7236) -> (w7237:dbl[])
            n1605 = call "CONEX_FUNCTIONAL_GLOBAL.vi"("Axis"=enum16{"X", "Y", "Z", "XY", "XZ", "YZ", "XYZ"}."Z", "Position"=w7237, "Command"=T23."REL MOVE") -> ()  [unwired: 6 in, 3 out]
          }
          frame Default {
          }
          frame "Insert" {
          }
          frame "Delete" {
          }
          frame "Home" {
          }
          frame "End" {
          }
          frame "Escape" {
          }
          frame "Help" {
          }
          frame "Pause" {
          }
          frame "ScrollLock" {
          }
          frame "F1" {
          }
          frame "F2" {
          }
          frame "F3" {
          }
          frame "F4" {
          }
          frame "F5" {
            n1606 = local read "Inject Top"() -> (w7242:bool)
            n1607 = Not(x=w7242) -> (.not. x?=w7241:bool)
            n1608 = property on="Inject Top" class="Bool (strict)"("Val(Sgnl)"=w7241) -> ()  [unwired: 2 in, 2 out]
          }
          frame "F6" {
          }
          frame "F7" {
          }
          frame "F8" {
          }
          frame "F9" {
            n1609 = local read "Trap 1 (ON/OFF)"() -> (w7244:bool)
            n1610 = Not(x=w7244) -> (.not. x?=w7243:bool)
            n1611 = property on="Trap 1 (ON/OFF)" class="Bool (strict)"("Val(Sgnl)"=w7243) -> ()  [unwired: 2 in, 2 out]
          }
          frame "F10" {
            n1612 = local read "Trap 2 (ON/OFF)"() -> (w7246:bool)
            n1613 = Not(x=w7246) -> (.not. x?=w7245:bool)
            n1614 = property on="Trap 2 (ON/OFF)" class="Bool (strict)"("Val(Sgnl)"=w7245) -> ()  [unwired: 2 in, 2 out]
          }
          frame "F11" {
            n1615 = local read "Sample Channel Flow"() -> (w7248:bool)
            n1616 = Not(x=w7248) -> (.not. x?=w7247:bool)
            n1617 = case shown="True" w7247 {
              frame False {
              }
              frame True {
                n1618 = property on="Inject Bottom" class="Bool (strict)"("Val(Sgnl)"=FALSE ("Value (Signaling)")) -> ()  [unwired: 2 in, 2 out]
                n1619 = property on="Inject Top" class="Bool (strict)"("Val(Sgnl)"=FALSE ("Value (Signaling)")) -> ()  [unwired: 2 in, 2 out]
              }
            }
            n1620 = property on="Sample Channel Flow" class="Bool (strict)"("Val(Sgnl)"=w7247) -> ()  [unwired: 2 in, 2 out]
          }
          frame "F12" {
            n1621 = local read "Use mouse to move stage\n(press mouse wheel to quit)"() -> (w7252:bool)
            n1622 = Not(x=w7252) -> (.not. x?=w7251:bool)
            n1623 = case shown="False" w7251 {
              frame False {
                n1624 = flat-sequence {
                  frame #0 {
                    n1625 = dll-call lib="user32.dll" fn="ShowCursor" label="Call Library Function"("Enable"=1) -> ()  [unwired: 3 in, 4 out]
                  }
                  frame #1 {
                    n1626 = Wait (ms)(milliseconds to wait=u32 1000) -> ()  [unwired: 1 out]
                  }
                }
                n1627 = property class="VI"() -> ("Panel"=w7254:refnum<vi>)  [unwired: 2 in, 2 out]
                n1628 = property class="Pnl"(reference=w7254) -> ("Panes[]"=w7255:refnum<vi>[])  [unwired: 1 in, 2 out]
                n1629 = for {
                  tunnel: w7255 -> [w7259] mode=indexing
                  tunnel: T47."Always On" ("Horizontal Scrollbar Visibility") -> [w7260]
                  n1630 = property class="Pane"(reference=w7259, "HorizScrollbarVisibility"=w7260) -> (reference out=w7258:refnum<vi>)  [unwired: 1 in, 1 out]
                  n1631 = property class="Pane"(reference=w7258, "VertScrollbarVisibility"=w7260) -> ()  [unwired: 1 in, 2 out]
                }
              }
              frame True {
                n1632 = property class="VI"() -> ("Panel"=w7262:refnum<vi>)  [unwired: 2 in, 2 out]
                n1633 = property class="Pnl"(reference=w7262) -> ("Panes[]"=w7263:refnum<vi>[])  [unwired: 1 in, 2 out]
                n1634 = flat-sequence {
                  frame #0 {
                    n1635 = dll-call lib="user32.dll" fn="ShowCursor" label="Call Library Function"("Enable"=0) -> ()  [unwired: 3 in, 4 out]
                  }
                  frame #1 {
                    n1636 = Wait (ms)(milliseconds to wait=u32 1000) -> ()  [unwired: 1 out]
                  }
                }
                n1637 = for {
                  tunnel: w7263 -> [w7268] mode=indexing
                  tunnel: T47."Always Off" ("Horizontal Scrollbar Visibility") -> [w7266]
                  n1638 = property class="Pane"(reference=w7268, "HorizScrollbarVisibility"=w7266) -> (reference out=w7267:refnum<vi>)  [unwired: 1 in, 1 out]
                  n1639 = property class="Pane"(reference=w7267, "VertScrollbarVisibility"=w7266) -> ()  [unwired: 1 in, 2 out]
                }
              }
            }
            n1640 = local write "Use mouse to move stage\n(press mouse wheel to quit)"(w7251) -> ()
          }
          frame "F13" {
          }
          frame "F14" {
          }
          frame "F15" {
          }
          frame "F16" {
          }
          frame "F17" {
          }
          frame "F18" {
          }
          frame "F19" {
          }
          frame "F20" {
          }
          frame "F21" {
          }
          frame "F22" {
          }
          frame "F23" {
          }
          frame "F24" {
          }
          frame "Play" {
          }
          frame "VolumeUp" {
          }
          frame "VolumeDown" {
          }
          frame "Mute" {
          }
          frame "Two Byte Char" {
          }
          frame "Break" {
          }
          frame "Clear" {
          }
          frame "NumLock" {
          }
          frame "Caps" {
          }
          frame "Opt" {
          }
          frame "Cmd" {
          }
          frame "Alt" {
          }
          frame "Ctrl" {
          }
          frame "Shift" {
          }
          frame "Return" {
          }
          frame "Enter" {
          }
          frame "ASCII" {
          }
        }
      }
      event "Read Cal": Value Change {
        w7270 = 1000.0 ("y")
        n1641 = event-data() -> ()  [unwired: 7 out]
        n1642 = local read "Save file name"() -> (w7295:path)
        n1643 = local write "Read Cal"(FALSE ("Read Cal")) -> ()
        n1644 = Strip Path(path=w7295) -> (stripped path=w7294:path)  [unwired: 1 out]
        n1645 = Path To String(path=w7294) -> (string=w7293:string)
        n1646 = Concatenate Strings(w7293, "\\current.cal" ("string")) -> (w7291:string)
        n1647 = String To Path(string=w7291) -> (path=w7290:path)
        n1648 = Open/Create/Replace File(file path (use dialog)=w7290, operation (0:open)=T25."open", access (0:read/write)=enum16{"read/write", "read-only", "write-only"}."read-only") -> (refnum out=w7298:refnum<file>, error out=w7284:errorcluster)  [unwired: 1 in, 3 out]
        n1649 = Deny Access(4:w7284, 7:w7298) -> (0:w7283:errorcluster, 3:w7289:refnum<file>)  [unwired: 1 out]
        n1650 = Read from Binary File(5:0.0, 8:w7283, 9:T39."big-endian, network order" ("byte order (0:big-endian, network order)"), 10:-1 ("count (1)"), 11:w7289) -> (0:w7282:errorcluster, 2:w7280:dbl[], 3:w7285:refnum<file>)  [unwired: 2 out]
        n1651 = Array To Cluster(array=w7280) -> (cluster=w7279:T50)
        n1652 = Unbundle(w7279) -> ("[0]"=w7278:dbl, "[1]"=w7277:dbl, "[2]"=w7276:dbl, "[3]"=w7275:dbl, "[4]"=w7274:dbl, "[5]"=w7273:dbl)
        n1653 = Close File(refnum=w7285, error in=w7282) -> (error out=→"Read cal error":errorcluster)  [unwired: 1 out]
        n1654 = Multiply(x=w7273, y=w7270) -> (x*y=w7271:dbl)
        n1655 = local write "T2 kappa_x (pN/nm)"(w7275) -> ()
        n1656 = local write "T1 kappa_x (pN/nm)"(w7276) -> ()
        n1657 = local write "T1 alpha_x (nm/V)"(w7278) -> ()
        n1658 = local write "T2 alpha_x (nm/V)"(w7277) -> ()
        n1659 = Multiply(x=w7274, y=w7270) -> (x*y=w7272:dbl)
        n1660 = local write "T1 offset_x (mV)"(w7272) -> ()
        n1661 = local write "T2 offset_x (mV)"(w7271) -> ()
      }
      event "Abort MCL Scan": Value Change {
        n1662 = event-data() -> ()  [unwired: 7 out]
        n1663 = local write "MCL Scanning"(FALSE ("MCL Scanning")) -> ()
        n1664 = xnode "Read/Write Control"("FPGA VI Reference In"=w7303, "error in"=w7302, "Abort scan (MCL)"="Abort MCL Scan") -> ("error out"=w7301:errorcluster)  [unwired: 1 out]
      }
      event "Update Count (MCL)": Value Change {
        n1665 = event-data() -> ()  [unwired: 7 out]
        n1666 = xnode "Read/Write Control"("FPGA VI Reference In"=w7345, "error in"=w7344, "MCL count"="Update Count (MCL)") -> ("error out"=w7343:errorcluster)  [unwired: 1 out]
      }
      event "Phase adjust (MCL)", "+ phase (MCL)", "- phase (MCL)": Value Change {
        n1667 = event-data() -> ()  [unwired: 7 out]
        n1668 = Negate(x="Phase adjust (MCL)") -> (-x=w7391:i16)
        n1669 = Select(t=w7391, s="- phase (MCL)", f="Phase adjust (MCL)") -> (s? t:f=w7389:i16)
        n1670 = Or(x="- phase (MCL)", y="+ phase (MCL)") -> (x .or. y?=w7384:bool)
        n1671 = xnode "Read/Write Control"("FPGA VI Reference In"=w7393, "error in"=w7392, "Phase count adjustment (MCL)"=w7389) -> ("FPGA VI Reference Out"=w7385:T20, "error out"=w7386:errorcluster)
        n1672 = xnode "Read/Write Control"("FPGA VI Reference In"=w7385, "error in"=w7386, "+ phase (MCL)"=w7384) -> ("error out"=w7383:errorcluster)  [unwired: 1 out]
      }
      event "Abort AOD Scan": Value Change {
        n1673 = event-data() -> ()  [unwired: 7 out]
        n1674 = xnode "Read/Write Control"("FPGA VI Reference In"=w7472, "error in"=w7471, "Abort scan"="Abort AOD Scan") -> ("error out"=w7470:errorcluster)  [unwired: 1 out]
      }
      event "Continuous AOD Scanning": Value Change {
        n1675 = event-data() -> ()  [unwired: 7 out]
        n1676 = xnode "Read/Write Control"("FPGA VI Reference In"=w7514, "error in"=w7513, "Cont. Scan"="Continuous AOD Scanning") -> ("error out"=w7512:errorcluster)  [unwired: 1 out]
      }
      event "Index": Value Change {
        n1677 = event-data() -> ()  [unwired: 7 out]
        n1678 = call "Create new save file.vi"("Insert"="", "Ext"=".dat" ("string"), "Index In"="Index") -> ("Path Out"=→"Save file name":path, "Index Out"=w7553:dbl)
        "Save index" <- w7553
        n1679 = local write "Index"(w7553) -> ()
      }
      event "AO1", "AO2": Value Change {
        w7568 = 10.0 ("y")
        w7567 = 32767.0 ("y")
        n1680 = event-data() -> ()  [unwired: 7 out]
        n1681 = local read "AO2"() -> (w7566:dbl)
        n1682 = local read "AO1"() -> (w7563:dbl)
        n1683 = Multiply(x=w7563, y=w7567) -> (x*y=w7562:dbl)
        n1684 = Multiply(x=w7566, y=w7567) -> (x*y=w7565:dbl)
        n1685 = Divide(x=w7562, y=w7568) -> (x/y=w7561:dbl)
        n1686 = Divide(x=w7565, y=w7568) -> (x/y=w7564:dbl)
        n1687 = To Word Integer(number=w7561) -> (16bit integer=w7569:i16)
        n1688 = To Word Integer(number=w7564) -> (16bit integer=w7570:i16)
        n1689 = xnode "Read/Write Control"("FPGA VI Reference In"=w7560, "error in"=w7559, "AO1"=w7569, "AO2"=w7570) -> ("error out"=w7558:errorcluster)  [unwired: 1 out]
      }
      event "Inject Top": Value Change {
        n1690 = event-data() -> ("NewVal"=w7630:bool)  [unwired: 6 out]
        n1691 = disable-structure shown="Enabled" {
          disable-tunnel: w7630 -> [_ w7675]
          disable-tunnel: w7629 -> [_ w7674]
          disable-tunnel: [_ w7673] -> w7628
          frame Disabled {
            n1692 = local read "Chemyx Syringe Pump Serial Port"() -> (w7631:refnum<visa-resource-name>)
            n1693 = local read "Pump write delay (ms)"() -> (w7632:dbl)
            n1694 = case shown="True" "Inject Top" {
              tunnel: w7632 -> [w7639 w7653]
              tunnel: w7631 -> [w7636 w7652]
              frame False {
                n1695 = flat-sequence {
                  tunnel: w7636 -> [w7640]
                  tunnel: [w7640] -> w7637
                  tunnel: w7639 -> [_]
                  tunnel: [w7643] -> w7638
                  tunnel: w7637 -> [w7643]
                  tunnel: w7638 -> [w7644]
                  tunnel: [w7644] -> w7634
                  tunnel: [w7646] -> w7635
                  tunnel: w7634 -> [w7646]
                  tunnel: w7635 -> [w7648]
                  frame #0 {
                    n1696 = call "Write to pump.vi"("string"="enter pump1", "VISA resource name"=w7640) -> ()  [unwired: 1 out]
                  }
                  frame #1 {
                    n1697 = Wait (ms)(milliseconds to wait="Pump pause delay (ms)") -> ()  [unwired: 1 out]
                  }
                  frame #2 {
                    n1698 = call "Write to pump.vi"("string"="stop", "VISA resource name"=w7644) -> ()  [unwired: 1 out]
                  }
                  frame #3 {
                    n1699 = Wait (ms)(milliseconds to wait=u32 500) -> ()  [unwired: 1 out]
                  }
                  frame #4 {
                    n1700 = call "Write to pump.vi"("string"="stop", "VISA resource name"=w7648) -> ()  [unwired: 1 out]
                  }
                }
              }
              frame True {
                n1701 = flat-sequence {
                  tunnel: w7652 -> [w7662]
                  tunnel: w7653 -> [w7657]
                  tunnel: w7653 -> [w7664]
                  tunnel: w7652 -> [w7665]
                  tunnel: [w7665] -> w7650
                  tunnel: [w7667] -> w7651
                  tunnel: w7650 -> [w7667]
                  tunnel: w7651 -> [w7669]
                  frame #0 {
                    n1702 = local read "All Pump Parameters"() -> (w7656:T5)
                    n1703 = Unbundle By Name(w7656) -> ("Pump 1"=w7663:T51)
                    n1704 = call "Set pump parameters.vi"("Pump write delay (ms)"=w7657, "Volume (uL)"="Ch 2 Inject Volume (uL)", "Rate (uL/h)"="Ch 1 Inject Rate (ul/h)", "Units"=4.0, "Pump #"=1.0, "Pump Parameters In"=w7663, "VISA resource name"=w7662) -> ("Pump Parameters Out"=w7655:T51)  [unwired: 3 in]
                    n1705 = Bundle By Name(cluster=w7656, "Pump 1"=w7655) -> (w7654:T5)
                    n1706 = local write "All Pump Parameters"(w7654) -> ()
                  }
                  frame #1 {
                    n1707 = Wait (ms)(milliseconds to wait=w7664) -> ()  [unwired: 1 out]
                  }
                  frame #2 {
                    n1708 = call "Write to pump.vi"("string"="start", "VISA resource name"=w7665) -> ()  [unwired: 1 out]
                  }
                  frame #3 {
                    n1709 = Wait (ms)(milliseconds to wait=u32 500) -> ()  [unwired: 1 out]
                  }
                  frame #4 {
                    n1710 = call "Write to pump.vi"("string"="start", "VISA resource name"=w7669) -> ()  [unwired: 1 out]
                  }
                }
              }
            }
          }
          frame Enabled {
            n1711 = call "hamilton_controller.vi"("error in"=w7674, "Open?"=w7675, "valve"=enum16{"A", "B", "C", "D", "ALL"}."D", "action"=T17."MOVE VALVE") -> ("error out"=w7673:errorcluster)  [unwired: 7 in]